vi "FlexMag - 23-03-2023.vi"() -> ()   [LabVIEW 2018] (continued)
                            }
                          }
                          frame #1 {
                            n17701 = while {
                              i -> [w22606]
                              stop <- w22602 stop-if-true
                              n17702 = Greater Or Equal?(x=w22606, y=200) -> (x >= y?=w22608:bool)
                              n17703 = case shown="True" w22608 {
                                frame False {
                                }
                                frame True {
                                n17704 = local write "ch1 pumpdown error"(TRUE ("ch1 pumpdown error")) -> ()
                                n17705 = local write "Warning Message"("CH1 PumpDown process  is canceled !\nCH1 PC GV couldn't be opened" ("Warning Message")) -> ()
                                }
                              }
                              n17706 = local read "ch1 pumpdown alg"() -> (w22605:bool)
                              n17707 = local read "ch1_pcgv_gui"() -> (w22601:bool)
                              n17708 = local read "abort ch1"() -> (w22603:bool)
                              n17709 = Wait Until Next ms Multiple(millisecond multiple=u32 200) -> ()  [unwired: 1 out]
                              n17710 = Not(x=w22605) -> (.not. x?=w22604:bool)
                              n17711 = Compound Arithmetic op=OR(w22601, w22603, w22604) -> (w22602:bool)
                            }
                          }
                        }
                      }
                      frame True {
                      }
                    }
                  }
                }
              }
              frame #20 {
                n17712 = local read "ch1 pumpdown alg"() -> (w22611:bool)
                n17713 = case shown="True" w22611 {
                  frame False {
                  }
                  frame True {
                    n17714 = local read "abort ch1"() -> (w22612:bool)
                    n17715 = case shown="False" w22612 {
                      frame False {
                        n17716 = local write "ch1 pc gv open led"(TRUE ("ch1 ch vbv close")) -> ()
                        n17717 = Wait (ms)(milliseconds to wait=u32 1000) -> ()  [unwired: 1 out]
                      }
                      frame True {
                      }
                    }
                  }
                }
              }
              frame #21 {
                # "ch pressure check"
                n17718 = local read "ch1 pumpdown alg"() -> (w22615:bool)
                n17719 = case shown="True" w22615 {
                  frame False {
                  }
                  frame True {
                    n17720 = local read "abort ch1"() -> (w22616:bool)
                    n17721 = case shown="False" w22616 {
                      frame False {
                        n17722 = while {
                          i -> [w22623]
                          stop <- w22627 stop-if-true
                          # "30 min"
                          n17723 = Greater?(x=w22623, y=9000) -> (0:w22620:bool)
                          n17724 = case shown="True" w22620 {
                            frame False {
                            }
                            frame True {
                              n17725 = local write "Warning Message"("CH1 PumpDown process  is canceled !\nCH1 CH Pressure couldn't be reached under 0.5 Torr" ("Warning Message")) -> ()
                              n17726 = local write "ch1 pumpdown error"(TRUE ("ch1 pumpdown error")) -> ()
                            }
                          }
                          n17727 = local read "ch1 ch pg torr"() -> (w22619:dbl)
                          n17728 = Less Or Equal?(x=w22619, y=0.5) -> (x <= y?=w22617:bool)
                          n17729 = case shown="True" w22617 {
                            tunnel: [FALSE TRUE] -> w22621
                            frame False {
                              n17730 = Wait Until Next ms Multiple(millisecond multiple=u32 200) -> ()  [unwired: 1 out]
                            }
                            frame True {
                            }
                          }
                          n17731 = local read "ch1 pumpdown alg"() -> (w22626:bool)
                          n17732 = local read "abort ch1"() -> (w22624:bool)
                          n17733 = Not(x=w22626) -> (.not. x?=w22625:bool)
                          n17734 = Compound Arithmetic op=OR(w22621, w22624, w22625) -> (w22627:bool)
                        }
                      }
                      frame True {
                      }
                    }
                  }
                }
              }
              frame #22 {
                n17735 = local read "ch1 pumpdown alg"() -> (w22633:bool)
                n17736 = case shown="True" w22633 {
                  frame False {
                  }
                  frame True {
                    n17737 = local read "abort ch1"() -> (w22634:bool)
                    n17738 = case shown="False" w22634 {
                      frame False {
                        n17739 = local write "ch1 ch press under 0.5 T led"(TRUE ("ch1 ch pressure led")) -> ()
                        n17740 = Wait (ms)(milliseconds to wait=u32 1000) -> ()  [unwired: 1 out]
                      }
                      frame True {
                      }
                    }
                  }
                }
              }
              frame #23 {
                # "ch 2 pressure check\nfor trns bp bv"
                n17741 = local read "ch1 pumpdown alg"() -> (w22637:bool)
                n17742 = case shown="True" w22637 {
                  frame False {
                  }
                  frame True {
                    n17743 = local read "abort ch1"() -> (w22638:bool)
                    n17744 = case shown="False" w22638 {
                      frame False {
                        n17745 = local read "ch2 ch pg torr"() -> (w22641:dbl)
                        n17746 = Less Or Equal?(x=w22641, y=0.5) -> (x <= y?=w22639:bool)
                        n17747 = case shown="True" w22639 {
                          frame False {
                          }
                          frame True {
                            n17748 = stacked-sequence {
                              frame #0 {
                                n17749 = while {
                                i -> [w22646]
                                stop <- w22650 stop-if-true
                                n17750 = Greater?(x=w22646, y=100) -> (0:w22643:bool)
                                n17751 = case shown="True" w22643 {
                                frame False {
                                }
                                frame True {
                                n17752 = local write "Warning Message"("CH1 PumpDown process  is canceled !\nCH1 Trns BP Left couldn't be opened" ("Warning Message")) -> ()
                                n17753 = local write "ch1 pumpdown error"(TRUE ("ch1 pumpdown error")) -> ()
                                }
                                }
                                n17754 = local read "CH1_Trns_BP_Left_DI"() -> (w22642:bool)
                                n17755 = case shown="False" w22642 {
                                tunnel: [FALSE TRUE] -> w22644
                                frame False {
                                n17756 = local write "CH1_Trns_BP_Left_DO"(TRUE ("CH1_Trns_BP_Left_DO")) -> ()
                                n17757 = Wait Until Next ms Multiple(millisecond multiple=u32 200) -> ()  [unwired: 1 out]
                                }
                                frame True {
                                }
                                }
                                n17758 = local read "ch1 pumpdown alg"() -> (w22649:bool)
                                n17759 = local read "abort ch1"() -> (w22647:bool)
                                n17760 = Not(x=w22649) -> (.not. x?=w22648:bool)
                                n17761 = Compound Arithmetic op=OR(w22644, w22647, w22648) -> (w22650:bool)
                                }
                              }
                              frame #1 {
                                n17762 = local read "ch1 pumpdown alg"() -> (w22657:bool)
                                n17763 = case shown="True" w22657 {
                                frame False {
                                }
                                frame True {
                                n17764 = local read "abort ch1"() -> (w22658:bool)
                                n17765 = case shown="False" w22658 {
                                frame False {
                                n17766 = local write "ch1 trns bp left open led"(TRUE ("ch1 tp start led")) -> ()
                                n17767 = local write "ch1_2 vacuum level"("VACUUM" ("ch3_4 vacuum level")) -> ()
                                n17768 = Wait (ms)(milliseconds to wait=u32 1000) -> ()  [unwired: 1 out]
                                }
                                frame True {
                                }
                                }
                                }
                                }
                              }
                              frame #2 {
                                n17769 = while {
                                i -> [w22664]
                                stop <- w22666 stop-if-true
                                n17770 = Wait Until Next ms Multiple(millisecond multiple=u32 200) -> ()  [unwired: 1 out]
                                n17771 = local read "ch1 pumpdown alg"() -> (w22667:bool)
                                n17772 = local read "abort ch1"() -> (w22669:bool)
                                n17773 = Greater?(x=w22664, y=100) -> (0:w22663:bool)
                                n17774 = Not(x=w22667) -> (.not. x?=w22668:bool)
                                n17775 = Compound Arithmetic op=OR(w22663, w22669, w22668) -> (w22666:bool)
                                }
                              }
                            }
                          }
                        }
                      }
                      frame True {
                      }
                    }
                  }
                }
              }
              frame #24 {
                # "ch pressure check"
                n17776 = local read "ch1 pumpdown alg"() -> (w22670:bool)
                n17777 = case shown="True" w22670 {
                  frame False {
                  }
                  frame True {
                    n17778 = local read "abort ch1"() -> (w22671:bool)
                    n17779 = case shown="False" w22671 {
                      frame False {
                        n17780 = while {
                          i -> [w22678]
                          stop <- w22682 stop-if-true
                          # "20 min"
                          n17781 = Greater?(x=w22678, y=6000) -> (0:w22675:bool)
                          n17782 = case shown="True" w22675 {
                            frame False {
                            }
                            frame True {
                              n17783 = local write "Warning Message"("CH1 PumpDown process  is canceled !\nCH1 CH Pressure couldn't be reached under 0.2 Torr" ("Warning Message")) -> ()
                              n17784 = local write "ch1 pumpdown error"(TRUE ("ch1 pumpdown error")) -> ()
                            }
                          }
                          n17785 = local read "ch1 ch pg torr"() -> (w22674:dbl)
                          n17786 = Less Or Equal?(x=w22674, y=0.5) -> (x <= y?=w22672:bool)
                          n17787 = case shown="False" w22672 {
                            tunnel: [FALSE TRUE] -> w22676
                            frame False {
                              n17788 = Wait Until Next ms Multiple(millisecond multiple=u32 200) -> ()  [unwired: 1 out]
                            }
                            frame True {
                            }
                          }
                          n17789 = local read "ch1 pumpdown alg"() -> (w22681:bool)
                          n17790 = local read "abort ch1"() -> (w22679:bool)
                          n17791 = Not(x=w22681) -> (.not. x?=w22680:bool)
                          n17792 = Compound Arithmetic op=OR(w22676, w22679, w22680) -> (w22682:bool)
                        }
                      }
                      frame True {
                      }
                    }
                  }
                }
              }
              frame #25 {
                # "tp start"
                n17793 = local read "ch1 pumpdown alg"() -> (w22688:bool)
                n17794 = case shown="True" w22688 {
                  frame False {
                  }
                  frame True {
                    n17795 = local read "abort ch1"() -> (w22689:bool)
                    n17796 = case shown="False" w22689 {
                      frame False {
                        n17797 = stacked-sequence {
                          frame #0 {
                            n17798 = flat-sequence {
                              frame #0 {
                                n17799 = local write "Tp1 auto start"(TRUE ("Tp1 auto start")) -> ()
                                n17800 = Wait (ms)(milliseconds to wait=u32 100) -> ()  [unwired: 1 out]
                              }
                              frame #1 {
                                n17801 = Wait (ms)(milliseconds to wait=u32 2000) -> ()  [unwired: 1 out]
                              }
                              frame #2 {
                                n17802 = disable-structure shown="Disabled" {
                                frame Disabled {
                                n17803 = local write "Tp1 Start initial"(TRUE ("Tp1 Start initial")) -> ()
                                }
                                frame Enabled {
                                }
                                }
                              }
                              frame #3 {
                                n17804 = Wait (ms)(milliseconds to wait=u32 2000) -> ()  [unwired: 1 out]
                              }
                              frame #4 {
                                n17805 = local write "Tp1 auto low speed"(TRUE ("Tp1 auto start")) -> ()
                                n17806 = Wait (ms)(milliseconds to wait=u32 100) -> ()  [unwired: 1 out]
                              }
                            }
                          }
                          frame #1 {
                            n17807 = while {
                              i -> [w22705]
                              stop <- w22699 stop-if-true
                              # "200 sec ?"
                              n17808 = Greater Or Equal?(x=w22705, y=1000) -> (x >= y?=w22698:bool)
                              n17809 = case shown="True" w22698 {
                                frame False {
                                }
                                frame True {
                                n17810 = local write "Warning Message"("CH1 PumpDown process  is canceled !\nCH1 TP couldn't be started" ("Warning Message")) -> ()
                                n17811 = local write "ch1 pumpdown error"(TRUE ("ch1 pumpdown error")) -> ()
                                }
                              }
                              n17812 = local read "ch1 pumpdown alg"() -> (w22702:bool)
                              n17813 = local read "ch1_tp_gui"() -> (w22697:bool)
                              n17814 = local read "abort ch1"() -> (w22700:bool)
                              n17815 = Not(x=w22702) -> (.not. x?=w22701:bool)
                              n17816 = Wait Until Next ms Multiple(millisecond multiple=u32 200) -> ()  [unwired: 1 out]
                              n17817 = Compound Arithmetic op=OR(w22697, w22700, w22701) -> (w22699:bool)
                            }
                          }
                        }
                      }
                      frame True {
                      }
                    }
                  }
                }
              }
              frame #26 {
                n17818 = local read "ch1 pumpdown alg"() -> (w22708:bool)
                n17819 = case shown="True" w22708 {
                  frame False {
                  }
                  frame True {
                    n17820 = local read "abort ch1"() -> (w22709:bool)
                    n17821 = case shown="False" w22709 {
                      frame False {
                        n17822 = local write "ch1 tp start led"(TRUE ("ch1 tp start led")) -> ()
                        n17823 = Wait (ms)(milliseconds to wait=u32 1000) -> ()  [unwired: 1 out]
                      }
                      frame True {
                      }
                    }
                  }
                }
              }
              frame #27 {
                n17824 = local read "ch1 pumpdown alg"() -> (w22712:bool)
                n17825 = case shown="True" w22712 {
                  frame False {
                  }
                  frame True {
                    n17826 = local read "abort ch1"() -> (w22713:bool)
                    n17827 = case shown="False" w22713 {
                      frame False {
                        n17828 = while {
                          i -> [w22720]
                          stop <- w22724 stop-if-true
                          # "30 min"
                          n17829 = Greater?(x=w22720, y=9000) -> (0:w22717:bool)
                          n17830 = case shown="True" w22717 {
                            frame False {
                            }
                            frame True {
                              n17831 = local write "Warning Message"("CH1 PumpDown process  is canceled !\nCH1 CH Pressure couldn't be reached under 0.01 Torr" ("Warning Message")) -> ()
                              n17832 = local write "ch1 pumpdown error"(TRUE ("ch1 pumpdown error")) -> ()
                            }
                          }
                          n17833 = local read "ch1 ch pg torr"() -> (w22716:dbl)
                          n17834 = Less Or Equal?(x=w22716, y=0.09) -> (x <= y?=w22714:bool)
                          n17835 = case shown="False" w22714 {
                            tunnel: [FALSE TRUE] -> w22718
                            frame False {
                              n17836 = Wait Until Next ms Multiple(millisecond multiple=u32 200) -> ()  [unwired: 1 out]
                            }
                            frame True {
                            }
                          }
                          n17837 = local read "ch1 pumpdown alg"() -> (w22723:bool)
                          n17838 = local read "abort ch1"() -> (w22721:bool)
                          n17839 = Not(x=w22723) -> (.not. x?=w22722:bool)
                          n17840 = Compound Arithmetic op=OR(w22718, w22721, w22722) -> (w22724:bool)
                        }
                      }
                      frame True {
                      }
                    }
                  }
                }
              }
              frame #28 {
                n17841 = local read "ch1 pumpdown alg"() -> (w22730:bool)
                n17842 = case shown="True" w22730 {
                  frame False {
                  }
                  frame True {
                    n17843 = local read "abort ch1"() -> (w22731:bool)
                    n17844 = case shown="False" w22731 {
                      frame False {
                        n17845 = local write "ch1 ch press under 0.01 T led"(TRUE ("ch1 pressure under 0.05 torr led")) -> ()
                        n17846 = Wait (ms)(milliseconds to wait=u32 1000) -> ()  [unwired: 1 out]
                      }
                      frame True {
                      }
                    }
                  }
                }
              }
              frame #29 {
                # "CC open"
                n17847 = local read "ch1 pumpdown alg"() -> (w22734:bool)
                n17848 = case shown="True" w22734 {
                  frame False {
                  }
                  frame True {
                    n17849 = local read "abort ch1"() -> (w22735:bool)
                    n17850 = case shown="False" w22735 {
                      frame False {
                        n17851 = stacked-sequence {
                          frame #0 {
                            n17852 = while {
                              i -> [w22740]
                              stop <- w22744 stop-if-true
                              n17853 = Greater?(x=w22740, y=200) -> (0:w22737:bool)
                              n17854 = case shown="True" w22737 {
                                frame False {
                                }
                                frame True {
                                n17855 = local write "Warning Message"("CH1 PumpDown process  is canceled !\nCH1 CC couldn't be opened" ("Warning Message")) -> ()
                                n17856 = local write "ch1 pumpdown error"(TRUE ("ch1 pumpdown error")) -> ()
                                }
                              }
                              n17857 = local read "CH1_CC_DI"() -> (w22736:bool)
                              n17858 = case shown="False" w22736 {
                                tunnel: [FALSE TRUE] -> w22738
                                frame False {
                                n17859 = Wait Until Next ms Multiple(millisecond multiple=u32 200) -> ()  [unwired: 1 out]
                                n17860 = local write "CH1_CC_DO"(TRUE ("CH1_CC_DO")) -> ()
                                }
                                frame True {
                                }
                              }
                              n17861 = local read "ch1 pumpdown alg"() -> (w22743:bool)
                              n17862 = local read "abort ch1"() -> (w22741:bool)
                              n17863 = Not(x=w22743) -> (.not. x?=w22742:bool)
                              n17864 = Compound Arithmetic op=OR(w22738, w22741, w22742) -> (w22744:bool)
                            }
                          }
                          frame #1 {
                            n17865 = while {
                              i -> [w22753]
                              stop <- w22755 stop-if-true
                              n17866 = local read "ch1 pumpdown alg"() -> (w22756:bool)
                              n17867 = local read "abort ch1"() -> (w22758:bool)
                              n17868 = Greater Or Equal?(x=w22753, y=300) -> (x >= y?=w22751:bool)
                              n17869 = Not(x=w22756) -> (.not. x?=w22757:bool)
                              n17870 = Compound Arithmetic op=OR(w22751, w22758, w22757) -> (w22755:bool)
                              n17871 = Wait Until Next ms Multiple(millisecond multiple=u32 200) -> ()  [unwired: 1 out]
                            }
                          }
                        }
                      }
                      frame True {
                      }
                    }
                  }
                }
              }
              frame #30 {
                n17872 = local read "ch1 pumpdown alg"() -> (w22759:bool)
                n17873 = case shown="True" w22759 {
                  frame False {
                  }
                  frame True {
                    n17874 = local read "abort ch1"() -> (w22760:bool)
                    n17875 = case shown="False" w22760 {
                      frame False {
                        n17876 = local write "ch1 cc open led"(TRUE ("ch1 ch cc open led")) -> ()
                        n17877 = Wait (ms)(milliseconds to wait=u32 1000) -> ()  [unwired: 1 out]
                      }
                      frame True {
                      }
                    }
                  }
                }
              }
              frame #31 {
                n17878 = local read "ch1 pumpdown alg"() -> (w22763:bool)
                n17879 = case shown="True" w22763 {
                  frame False {
                  }
                  frame True {
                    n17880 = local read "abort ch1"() -> (w22764:bool)
                    n17881 = case shown="False" w22764 {
                      frame False {
                        n17882 = while {
                          i -> [w22775]
                          stop <- w22779 stop-if-true
                          # "60 min"
                          n17883 = Multiply(x=27000 ("y"), y=3) -> (x*y=w22765:i32)
                          n17884 = Greater?(x=w22775, y=w22765) -> (0:w22773:bool)
                          n17885 = case shown="True" w22773 {
                            frame False {
                            }
                            frame True {
                              n17886 = local write "Warning Message"("CH1 PumpDown process  is canceled !\nCH1 CH Pressure couldn't be reached to desired pressure" ("Warning Message")) -> ()
                              n17887 = local write "ch1 pumpdown error"(TRUE ("ch1 pumpdown error")) -> ()
                            }
                          }
                          n17888 = local read "ch1 cc torr"() -> (w22772:dbl)
                          n17889 = Multiply(x=0.75, y="ch1 desired pressure") -> (x*y=w22769:dbl)
                          n17890 = Less Or Equal?(x=w22772, y=w22769) -> (x <= y?=w22771:bool)
                          n17891 = case shown="False" w22771 {
                            tunnel: [FALSE TRUE] -> w22774
                            frame False {
                              n17892 = Wait Until Next ms Multiple(millisecond multiple=u32 200) -> ()  [unwired: 1 out]
                            }
                            frame True {
                            }
                          }
                          n17893 = local read "ch1 pumpdown alg"() -> (w22778:bool)
                          n17894 = local read "abort ch1"() -> (w22776:bool)
                          n17895 = Not(x=w22778) -> (.not. x?=w22777:bool)
                          n17896 = Compound Arithmetic op=OR(w22774, w22776, w22777) -> (w22779:bool)
                        }
                      }
                      frame True {
                      }
                    }
                  }
                }
              }
              frame #32 {
                n17897 = local read "ch1 pumpdown alg"() -> (w22785:bool)
                n17898 = case shown="True" w22785 {
                  frame False {
                  }
                  frame True {
                    n17899 = local read "abort ch1"() -> (w22786:bool)
                    n17900 = case shown="False" w22786 {
                      frame False {
                        n17901 = local write "ch1 desired pressure led"(TRUE ("ch1 pumdown completed led")) -> ()
                        n17902 = Wait (ms)(milliseconds to wait=u32 1000) -> ()  [unwired: 1 out]
                      }
                      frame True {
                      }
                    }
                  }
                }
              }
              frame #33 {
                n17903 = local read "ch1 pumpdown alg"() -> (w22789:bool)
                n17904 = case shown="True" w22789 {
                  frame False {
                  }
                  frame True {
                    n17905 = local read "abort ch1"() -> (w22790:bool)
                    n17906 = case shown="False" w22790 {
                      frame False {
                        w22792 = TRUE ("Buzzer DO")
                        n17907 = local write "Buzzer DO"(w22792) -> ()
                        n17908 = local write "CH1_BG_BV_DO"(TRUE ("CH1_BG_BV_DO")) -> ()
                        n17909 = local write "ch1 pd completed led"(w22792) -> ()
                        n17910 = Wait (ms)(milliseconds to wait=u32 3000) -> ()  [unwired: 1 out]
                        n17911 = local write "System Status"("CH1 PUMPDOWN PROCESS COMPLETED" ("System Status")) -> ()
                      }
                      frame True {
                      }
                    }
                  }
                }
              }
              frame #34 {
                n17912 = local read "ch1 pumpdown alg"() -> (w22795:bool)
                n17913 = case shown="True" w22795 {
                  frame False {
                  }
                  frame True {
                    n17914 = local read "abort ch1"() -> (w22796:bool)
                    n17915 = case shown="False" w22796 {
                      frame False {
                        w22798 = FALSE ("Buzzer DO")
                        n17916 = local write "Buzzer DO"(w22798) -> ()
                        n17917 = local write "ch1 pumpdown alg"(w22798) -> ()
                        n17918 = local write "Pump Down CH1"(w22798) -> ()
                        n17919 = Wait (ms)(milliseconds to wait=u32 3000) -> ()  [unwired: 1 out]
                        n17920 = local write "System Status"("SEMI-AUTOMATIC MODE " ("System Status")) -> ()
                      }
                      frame True {
                      }
                    }
                  }
                }
              }
            }
          }
          frame True {
          }
        }
      }
    }
    n17921 = case shown="True" "ch1 shutdown alg" {
      frame False {
      }
      frame True {
        n17922 = local read "abort ch1"() -> (w22019:bool)
        n17923 = case shown="False" w22019 {
          frame False {
            n17924 = stacked-sequence {
              frame #0 {
                n17925 = stacked-sequence {
                  frame #0 {
                    n17926 = local write "ch1 vent?"(FALSE ("ch1 vent?")) -> ()
                    n17927 = Wait (ms)(milliseconds to wait=u32 1000) -> ()  [unwired: 1 out]
                  }
                  frame #1 {
                    n17928 = local write "System Status"("CH1 SHUTDOWN PROCESS IN PROGRESS" ("System Status")) -> ()
                  }
                  frame #2 {
                    n17929 = Two Button Dialog(message="Do you want to Vent CH1 ?", 1:"No, SHUTDOWN only" ("F button name (\"Cancel\")"), 2:"Yes, VENT! CH1" ("T button name (\"OK\")")) -> (T button?=w22023:bool)
                    "ch1 vent?" <- w22023
                    n17930 = case shown="True" w22023 {
                      frame False {
                      }
                      frame True {
                        n17931 = local write "CH2_Trns_BP_Right_DO"(FALSE ("CH2_Trns_BP_Right_DO")) -> ()
                      }
                    }
                  }
                }
              }
              frame #1 {
                # "ATMs close"
                n17932 = local read "ch1 shutdown alg"() -> (w22028:bool)
                n17933 = case shown="True" w22028 {
                  frame False {
                  }
                  frame True {
                    n17934 = local read "abort ch1"() -> (w22029:bool)
                    n17935 = case shown="False" w22029 {
                      frame False {
                        w22030 = FALSE ("CH1_PL_ATM_DO")
                        n17936 = local write "CH1_PL_ATM_DO"(w22030) -> ()
                        n17937 = local write "CH1_CH_ATM_DO"(w22030) -> ()
                        n17938 = Wait (ms)(milliseconds to wait=u32 3000) -> ()  [unwired: 1 out]
                      }
                      frame True {
                      }
                    }
                  }
                }
              }
              frame #2 {
                n17939 = local read "ch1 shutdown alg"() -> (w22032:bool)
                n17940 = case shown="True" w22032 {
                  frame False {
                  }
                  frame True {
                    n17941 = local read "abort ch1"() -> (w22033:bool)
                    n17942 = case shown="False" w22033 {
                      frame False {
                        n17943 = local write "ch1 sd atms close led"(TRUE ("ch1 sd cc close led")) -> ()
                        n17944 = Wait (ms)(milliseconds to wait=u32 1000) -> ()  [unwired: 1 out]
                      }
                      frame True {
                      }
                    }
                  }
                }
              }
              frame #3 {
                # "CC close"
                n17945 = local read "ch1 shutdown alg"() -> (w22036:bool)
                n17946 = case shown="True" w22036 {
                  frame False {
                  }
                  frame True {
                    n17947 = local read "abort ch1"() -> (w22037:bool)
                    n17948 = case shown="False" w22037 {
                      frame False {
                        n17949 = while {
                          i -> [w22042]
                          stop <- w22046 stop-if-true
                          n17950 = Greater?(x=w22042, y=100) -> (0:w22039:bool)
                          n17951 = case shown="True" w22039 {
                            frame False {
                            }
                            frame True {
                              n17952 = local write "Warning Message"("CH1 ShutDown process  is canceled !\nCH1 CC couldn't be closed" ("Warning Message")) -> ()
                              n17953 = local write "ch1 shutdown error"(TRUE ("ch1 pumpdown error")) -> ()
                            }
                          }
                          n17954 = local read "CH1_CC_DI"() -> (w22038:bool)
                          n17955 = case shown="True" w22038 {
                            tunnel: [TRUE FALSE] -> w22040
                            frame False {
                            }
                            frame True {
                              n17956 = Wait Until Next ms Multiple(millisecond multiple=u32 200) -> ()  [unwired: 1 out]
                              n17957 = local write "CH1_CC_DO"(FALSE ("CH1_CC_DO")) -> ()
                            }
                          }
                          n17958 = local read "ch1 shutdown alg"() -> (w22045:bool)
                          n17959 = local read "abort ch1"() -> (w22043:bool)
                          n17960 = Not(x=w22045) -> (.not. x?=w22044:bool)
                          n17961 = Compound Arithmetic op=OR(w22040, w22043, w22044) -> (w22046:bool)
                        }
                      }
                      frame True {
                      }
                    }
                  }
                }
              }
              frame #4 {
                n17962 = local read "ch1 shutdown alg"() -> (w22053:bool)
                n17963 = case shown="True" w22053 {
                  frame False {
                  }
                  frame True {
                    n17964 = local read "abort ch1"() -> (w22054:bool)
                    n17965 = case shown="False" w22054 {
                      frame False {
                        n17966 = local write "ch1 sd cc close led"(TRUE ("ch1 sd cc close led")) -> ()
                        n17967 = Wait (ms)(milliseconds to wait=u32 1000) -> ()  [unwired: 1 out]
                      }
                      frame True {
                      }
                    }
                  }
                }
              }
              frame #5 {
                # "bg bv close"
                n17968 = local read "ch1 shutdown alg"() -> (w22057:bool)
                n17969 = case shown="True" w22057 {
                  frame False {
                  }
                  frame True {
                    n17970 = local read "abort ch1"() -> (w22058:bool)
                    n17971 = case shown="False" w22058 {
                      frame False {
                        n17972 = while {
                          i -> [w22063]
                          stop <- w22067 stop-if-true
                          n17973 = Greater?(x=w22063, y=100) -> (0:w22060:bool)
                          n17974 = case shown="True" w22060 {
                            frame False {
                            }
                            frame True {
                              n17975 = local write "Warning Message"("CH1 ShutDown process  is canceled !\nCH1 BG BV couldn't be closed" ("Warning Message")) -> ()
                              n17976 = local write "ch1 shutdown error"(TRUE ("ch1 pumpdown error")) -> ()
                            }
                          }
                          n17977 = local read "CH1_BG_BV_DI"() -> (w22059:bool)
                          n17978 = case shown="True" w22059 {
                            tunnel: [TRUE FALSE] -> w22061
                            frame False {
                            }
                            frame True {
                              n17979 = Wait Until Next ms Multiple(millisecond multiple=u32 200) -> ()  [unwired: 1 out]
                              n17980 = local write "CH1_BG_BV_DO"(FALSE ("CH1_CC_DO")) -> ()
                            }
                          }
                          n17981 = local read "ch1 shutdown alg"() -> (w22066:bool)
                          n17982 = local read "abort ch1"() -> (w22064:bool)
                          n17983 = Not(x=w22066) -> (.not. x?=w22065:bool)
                          n17984 = Compound Arithmetic op=OR(w22061, w22064, w22065) -> (w22067:bool)
                        }
                      }
                      frame True {
                      }
                    }
                  }
                }
              }
              frame #6 {
                n17985 = local read "ch1 shutdown alg"() -> (w22074:bool)
                n17986 = case shown="True" w22074 {
                  frame False {
                  }
                  frame True {
                    n17987 = local read "abort ch1"() -> (w22075:bool)
                    n17988 = case shown="False" w22075 {
                      frame False {
                        n17989 = local write "ch1 sd bg bv close led"(TRUE ("ch1 sd cc close led")) -> ()
                        n17990 = Wait (ms)(milliseconds to wait=u32 1000) -> ()  [unwired: 1 out]
                      }
                      frame True {
                      }
                    }
                  }
                }
              }
              frame #7 {
                # "TP stop"
                n17991 = local read "ch1 shutdown alg"() -> (w22078:bool)
                n17992 = case shown="True" w22078 {
                  frame False {
                  }
                  frame True {
                    n17993 = local read "abort ch1"() -> (w22079:bool)
                    n17994 = case shown="False" w22079 {
                      frame False {
                        n17995 = stacked-sequence {
                          frame #0 {
                            n17996 = flat-sequence {
                              frame #0 {
                                n17997 = local write "Tp1 auto stop"(TRUE ("Tp1 auto stop")) -> ()
                                n17998 = Wait (ms)(milliseconds to wait=u32 100) -> ()  [unwired: 1 out]
                              }
                              frame #1 {
                                n17999 = Wait (ms)(milliseconds to wait=u32 5000) -> ()  [unwired: 1 out]
                              }
                              frame #2 {
                                n18000 = local write "Tp1 auto stop"(TRUE ("Tp1 auto stop")) -> ()
                                n18001 = Wait (ms)(milliseconds to wait=u32 100) -> ()  [unwired: 1 out]
                              }
                            }
                          }
                          frame #1 {
                            n18002 = while {
                              i -> [w22096]
                              stop <- w22091 stop-if-true
                              n18003 = Multiply(x=3000 ("y"), y=5) -> (x*y=w22085:i32)
                              n18004 = Greater Or Equal?(x=w22096, y=w22085) -> (x >= y?=w22090:bool)
                              n18005 = case shown="True" w22090 {
                                frame False {
                                }
                                frame True {
                                n18006 = local write "Warning Message"("CH1 ShutDown process  is canceled !\nCH1 TP couldn't be stopped" ("Warning Message")) -> ()
                                n18007 = local write "ch1 shutdown error"(TRUE ("ch1 pumpdown error")) -> ()
                                }
                              }
                              n18008 = local read "ch1 shutdown alg"() -> (w22094:bool)
                              n18009 = local read "ch1_tp_gui"() -> (w22089:bool)
                              n18010 = local read "abort ch1"() -> (w22092:bool)
                              n18011 = Not(x=w22089) -> (.not. x?=w22088:bool)
                              n18012 = Not(x=w22094) -> (.not. x?=w22093:bool)
                              n18013 = Wait Until Next ms Multiple(millisecond multiple=u32 200) -> ()  [unwired: 1 out]
                              n18014 = Compound Arithmetic op=OR(w22088, w22092, w22093) -> (w22091:bool)
                            }
                          }
                        }
                      }
                      frame True {
                      }
                    }
                  }
                }
              }
              frame #8 {
                n18015 = local read "ch1 shutdown alg"() -> (w22099:bool)
                n18016 = case shown="True" w22099 {
                  frame False {
                  }
                  frame True {
                    n18017 = local read "abort ch1"() -> (w22100:bool)
                    n18018 = case shown="False" w22100 {
                      frame False {
                        n18019 = local write "ch1 sd tp stop led"(TRUE ("ch1 sd cc close led")) -> ()
                        n18020 = Wait (ms)(milliseconds to wait=u32 1000) -> ()  [unwired: 1 out]
                      }
                      frame True {
                      }
                    }
                  }
                }
              }
              frame #9 {
                # "tp bv close"
                n18021 = local read "ch1 shutdown alg"() -> (w22103:bool)
                n18022 = case shown="True" w22103 {
                  frame False {
                  }
                  frame True {
                    n18023 = local read "abort ch1"() -> (w22104:bool)
                    n18024 = case shown="False" w22104 {
                      frame False {
                        n18025 = while {
                          i -> [w22109]
                          stop <- w22113 stop-if-true
                          n18026 = Greater?(x=w22109, y=100) -> (0:w22106:bool)
                          n18027 = case shown="True" w22106 {
                            frame False {
                            }
                            frame True {
                              n18028 = local write "Warning Message"("CH1 ShutDown process  is canceled !\nCH1 TP BV couldn't be closed" ("Warning Message")) -> ()
                              n18029 = local write "ch1 shutdown error"(TRUE ("ch1 pumpdown error")) -> ()
                            }
                          }
                          n18030 = local read "CH1_TP_BV_DI"() -> (w22105:bool)
                          n18031 = case shown="True" w22105 {
                            tunnel: [TRUE FALSE] -> w22107
                            frame False {
                            }
                            frame True {
                              n18032 = Wait Until Next ms Multiple(millisecond multiple=u32 200) -> ()  [unwired: 1 out]
                              n18033 = local write "CH1_TP_BV_DO"(FALSE ("CH1_CC_DO")) -> ()
                            }
                          }
                          n18034 = local read "ch1 shutdown alg"() -> (w22112:bool)
                          n18035 = local read "abort ch1"() -> (w22110:bool)
                          n18036 = Not(x=w22112) -> (.not. x?=w22111:bool)
                          n18037 = Compound Arithmetic op=OR(w22107, w22110, w22111) -> (w22113:bool)
                        }
                      }
                      frame True {
                      }
                    }
                  }
                }
              }
              frame #10 {
                n18038 = local read "ch1 shutdown alg"() -> (w22120:bool)
                n18039 = case shown="True" w22120 {
                  frame False {
                  }
                  frame True {
                    n18040 = local read "abort ch1"() -> (w22121:bool)
                    n18041 = case shown="False" w22121 {
                      frame False {
                        n18042 = local write "ch1 sd tp bv close led"(TRUE ("ch1 sd cc close led")) -> ()
                        n18043 = Wait (ms)(milliseconds to wait=u32 1000) -> ()  [unwired: 1 out]
                      }
                      frame True {
                      }
                    }
                  }
                }
              }
              frame #11 {
                # "mp stop"
                n18044 = local read "ch1 shutdown alg"() -> (w22124:bool)
                n18045 = case shown="True" w22124 {
                  frame False {
                  }
                  frame True {
                    n18046 = local read "abort ch1"() -> (w22125:bool)
                    n18047 = case shown="False" w22125 {
                      frame False {
                        n18048 = while {
                          i -> [w22130]
                          stop <- w22134 stop-if-true
                          n18049 = Greater?(x=w22130, y=100) -> (0:w22127:bool)
                          n18050 = case shown="True" w22127 {
                            frame False {
                            }
                            frame True {
                              n18051 = local write "Warning Message"("CH1 ShutDown process  is canceled !\nCH1 MP couldn't be stopped" ("Warning Message")) -> ()
                              n18052 = local write "ch1 shutdown error"(TRUE ("ch1 pumpdown error")) -> ()
                            }
                          }
                          n18053 = local read "CH1_MP_DI"() -> (w22126:bool)
                          n18054 = case shown="True" w22126 {
                            tunnel: [TRUE FALSE] -> w22128
                            frame False {
                            }
                            frame True {
                              n18055 = Wait Until Next ms Multiple(millisecond multiple=u32 200) -> ()  [unwired: 1 out]
                              n18056 = local write "CH1_MP_DO"(FALSE ("CH1_CC_DO")) -> ()
                            }
                          }
                          n18057 = local read "ch1 shutdown alg"() -> (w22133:bool)
                          n18058 = local read "abort ch1"() -> (w22131:bool)
                          n18059 = Not(x=w22133) -> (.not. x?=w22132:bool)
                          n18060 = Compound Arithmetic op=OR(w22128, w22131, w22132) -> (w22134:bool)
                        }
                      }
                      frame True {
                      }
                    }
                  }
                }
              }
              frame #12 {
                n18061 = local read "ch1 shutdown alg"() -> (w22141:bool)
                n18062 = case shown="True" w22141 {
                  frame False {
                  }
                  frame True {
                    n18063 = local read "abort ch1"() -> (w22142:bool)
                    n18064 = case shown="False" w22142 {
                      frame False {
                        n18065 = local write "ch1 sd mp stop led"(TRUE ("ch1 sd cc close led")) -> ()
                        n18066 = Wait (ms)(milliseconds to wait=u32 1000) -> ()  [unwired: 1 out]
                      }
                      frame True {
                      }
                    }
                  }
                }
              }
              frame #13 {
                # "pl vbv open"
                n18067 = local read "ch1 shutdown alg"() -> (w22145:bool)
                n18068 = case shown="True" w22145 {
                  frame False {
                  }
                  frame True {
                    n18069 = local read "abort ch1"() -> (w22146:bool)
                    n18070 = case shown="False" w22146 {
                      frame False {
                        n18071 = while {
                          i -> [w22151]
                          stop <- w22155 stop-if-true
                          n18072 = Greater?(x=w22151, y=100) -> (0:w22148:bool)
                          n18073 = case shown="True" w22148 {
                            frame False {
                            }
                            frame True {
                              n18074 = local write "Warning Message"("CH1 ShutDown process  is canceled !\nCH1 PL VBV couldn't be opened" ("Warning Message")) -> ()
                              n18075 = local write "ch1 shutdown error"(TRUE ("ch1 pumpdown error")) -> ()
                            }
                          }
                          n18076 = local read "CH1_PL_VBV_DI"() -> (w22147:bool)
                          n18077 = case shown="False" w22147 {
                            tunnel: [FALSE TRUE] -> w22149
                            frame False {
                              n18078 = Wait Until Next ms Multiple(millisecond multiple=u32 200) -> ()  [unwired: 1 out]
                              n18079 = local write "CH1_PL_VBV_DO"(TRUE ("CH1_CC_DO")) -> ()
                            }
                            frame True {
                            }
                          }
                          n18080 = local read "ch1 shutdown alg"() -> (w22154:bool)
                          n18081 = local read "abort ch1"() -> (w22152:bool)
                          n18082 = Not(x=w22154) -> (.not. x?=w22153:bool)
                          n18083 = Compound Arithmetic op=OR(w22149, w22152, w22153) -> (w22155:bool)
                        }
                      }
                      frame True {
                      }
                    }
                  }
                }
              }
              frame #14 {
                n18084 = local read "ch1 shutdown alg"() -> (w22162:bool)
                n18085 = case shown="True" w22162 {
                  frame False {
                  }
                  frame True {
                    n18086 = local read "abort ch1"() -> (w22163:bool)
                    n18087 = case shown="False" w22163 {
                      frame False {
                        n18088 = local write "ch1 sd pl vbv open led"(TRUE ("ch1 sd cc close led")) -> ()
                        n18089 = Wait (ms)(milliseconds to wait=u32 1000) -> ()  [unwired: 1 out]
                      }
                      frame True {
                      }
                    }
                  }
                }
              }
              frame #15 {
                n18090 = local read "ch1 shutdown alg"() -> (w22166:bool)
                n18091 = case shown="True" w22166 {
                  frame False {
                  }
                  frame True {
                    n18092 = local read "abort ch1"() -> (w22167:bool)
                    n18093 = case shown="False" w22167 {
                      frame False {
                        n18094 = local read "ch1 vent?"() -> (w22168:bool)
                        n18095 = case shown="True" w22168 {
                          frame False {
                            n18096 = stacked-sequence {
                              frame #0 {
                                n18097 = local read "ch1 shutdown alg"() -> (w22169:bool)
                                n18098 = case shown="True" w22169 {
                                frame False {
                                }
                                frame True {
                                n18099 = flat-sequence {
                                frame #0 {
                                n18100 = local write "pcgv1 auto close"(TRUE ("pcgv1 auto open")) -> ()
                                }
                                frame #1 {
                                n18101 = Wait (ms)(milliseconds to wait=u32 2000) -> ()  [unwired: 1 out]
                                }
                                frame #2 {
                                n18102 = local write "pcgv1 auto close"(TRUE ("pcgv1 auto open")) -> ()
                                }
                                }
                                }
                                }
                              }
                              frame #1 {
                                n18103 = while {
                                i -> [w22180]
                                stop <- w22176 stop-if-true
                                n18104 = Greater Or Equal?(x=w22180, y=200) -> (x >= y?=w22182:bool)
                                n18105 = case shown="True" w22182 {
                                frame False {
                                }
                                frame True {
                                n18106 = local write "ch1 shutdown error"(TRUE ("ch1 pumpdown error")) -> ()
                                n18107 = local write "Warning Message"("CH1 ShutDown process  is canceled !\nCH1 PC GV couldn't be closed" ("Warning Message")) -> ()
                                }
                                }
                                n18108 = local read "ch1_pcgv_gui"() -> (w22173:bool)
                                n18109 = local read "abort ch1"() -> (w22177:bool)
                                n18110 = local read "ch1 shutdown alg"() -> (w22179:bool)
                                n18111 = Wait Until Next ms Multiple(millisecond multiple=u32 200) -> ()  [unwired: 1 out]
                                n18112 = Not(x=w22173) -> (.not. x?=w22174:bool)
                                n18113 = Not(x=w22179) -> (.not. x?=w22178:bool)
                                n18114 = Compound Arithmetic op=OR(w22174, w22177, w22178) -> (w22176:bool)
                                }
                              }
                            }
                          }
                          frame True {
                            n18115 = stacked-sequence {
                              frame #0 {
                                n18116 = local read "ch1 shutdown alg"() -> (w22185:bool)
                                n18117 = case shown="True" w22185 {
                                frame False {
                                }
                                frame True {
                                n18118 = flat-sequence {
                                frame #0 {
                                n18119 = local write "pcgv1 auto open"(TRUE ("pcgv1 auto open")) -> ()
                                }
                                frame #1 {
                                n18120 = Wait (ms)(milliseconds to wait=u32 2000) -> ()  [unwired: 1 out]
                                }
                                frame #2 {
                                n18121 = local write "pcgv1 auto open"(TRUE ("pcgv1 auto open")) -> ()
                                }
                                }
                                }
                                }
                              }
                              frame #1 {
                                n18122 = while {
                                i -> [w22195]
                                stop <- w22191 stop-if-true
                                n18123 = Greater Or Equal?(x=w22195, y=200) -> (x >= y?=w22197:bool)
                                n18124 = case shown="True" w22197 {
                                frame False {
                                }
                                frame True {
                                n18125 = local write "ch1 shutdown error"(TRUE ("ch1 pumpdown error")) -> ()
                                n18126 = local write "Warning Message"("CH1 ShutDown process  is canceled !\nCH1 PC GV couldn't be opened" ("Warning Message")) -> ()
                                }
                                }
                                n18127 = local read "ch1 shutdown alg"() -> (w22194:bool)
                                n18128 = local read "ch1_pcgv_gui"() -> (w22190:bool)